vi "make 2D gaussian.vi"(9 "A":dbl=10.0, 10 "w":dbl=15.0) -> (0 "error out":errorcluster, 3 "LASER Pointing SYSTEM":dbl[][](graph))   [LabVIEW 2013]
uses:
  Interface/Non-General/BELLA/VIremote/VIremote.llb/VIremoteFunction.ctl
panel:
  in  "Next Button":bool
  in  "Previous Button":bool
  in  "Down Button":bool
  in  "Up Target":bool
  in  "error IO":errorcluster
  in  "Fire":bool
  out "Cursor.Cursor Position:Cursor Y":dbl
  out "Cursor.Cursor Position:Cursor X":dbl
  in  "Down":bool
  in  "Up":bool
  in  "Vertical":dbl
  in  "Right":bool
  in  "Left":bool
  in  "stop":bool
  in  "Horizontal":dbl
  out "#pix":dbl
  in  "No spot sizes 2":dbl=50.0 format="%.3f"
  out "x0":dbl=50.0
  in  "Ring":u16(ring)
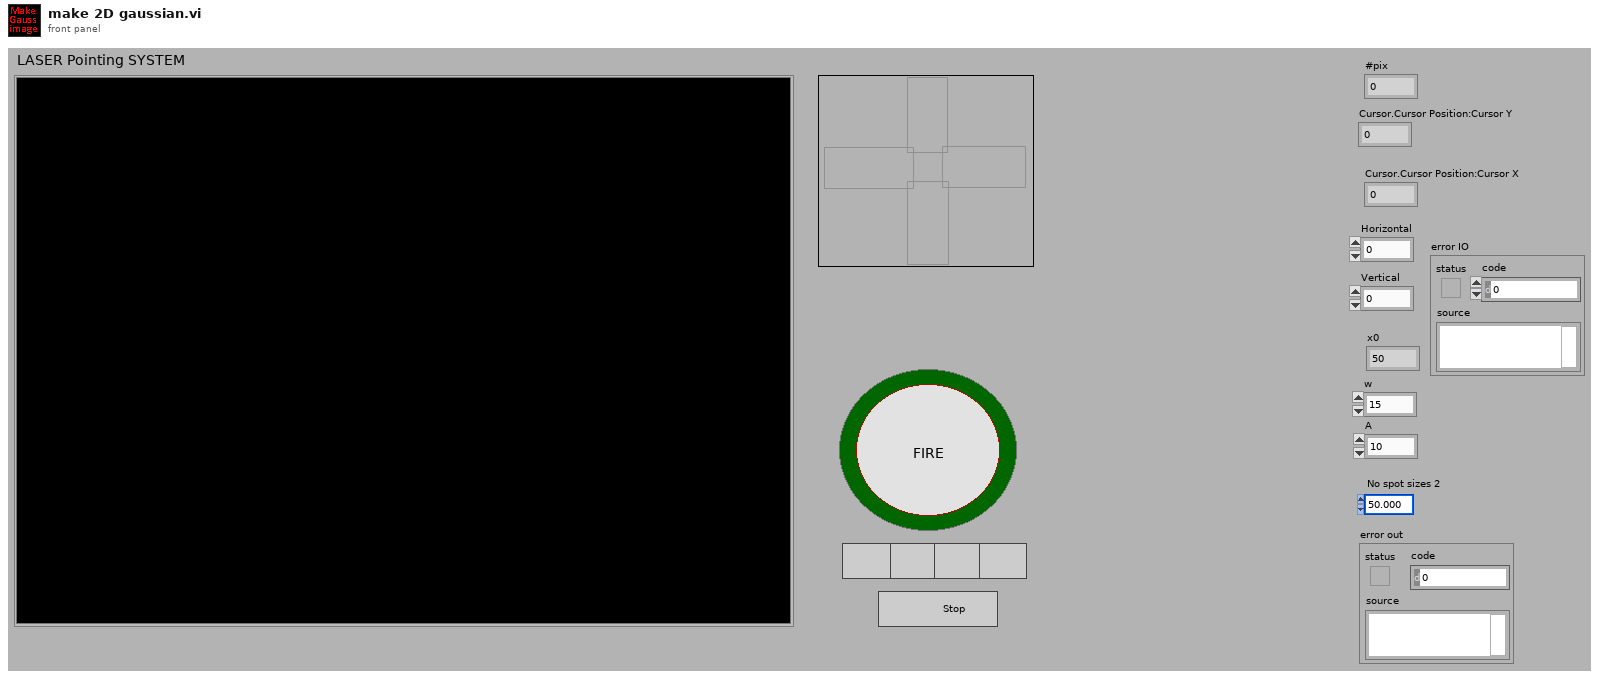
[diagram p1: front panel]
types:
  T1 = typedef "VIremoteFunction.ctl" = enum16{"Do nothing", "Stop controller", "Close this connection", "Show info panel", "Set VI to control", "Set Accelerometer freq (Hz)", "Show Alert message", "Start Sound Input", "Stop Sound Input", "Set Volume (0-100)", "Set sound output Speaker", "Set sound output Receiver", "Play Sound", "Repeat Sound", "Stop Sound", "Pause Sound", "Resume Sound", "Set panel width of caller (320 or 480)", "Set Panel Size to Portrait", "Set Panel Size to Landscape", "Set Panel Size as Current Orientation", "Allow all UI Orientations", "Send user notification", "Disable Scrolling", "Normal Scrolling", "Page Scrolling", "Set Scroll Offset", "Page Indicator Position"}
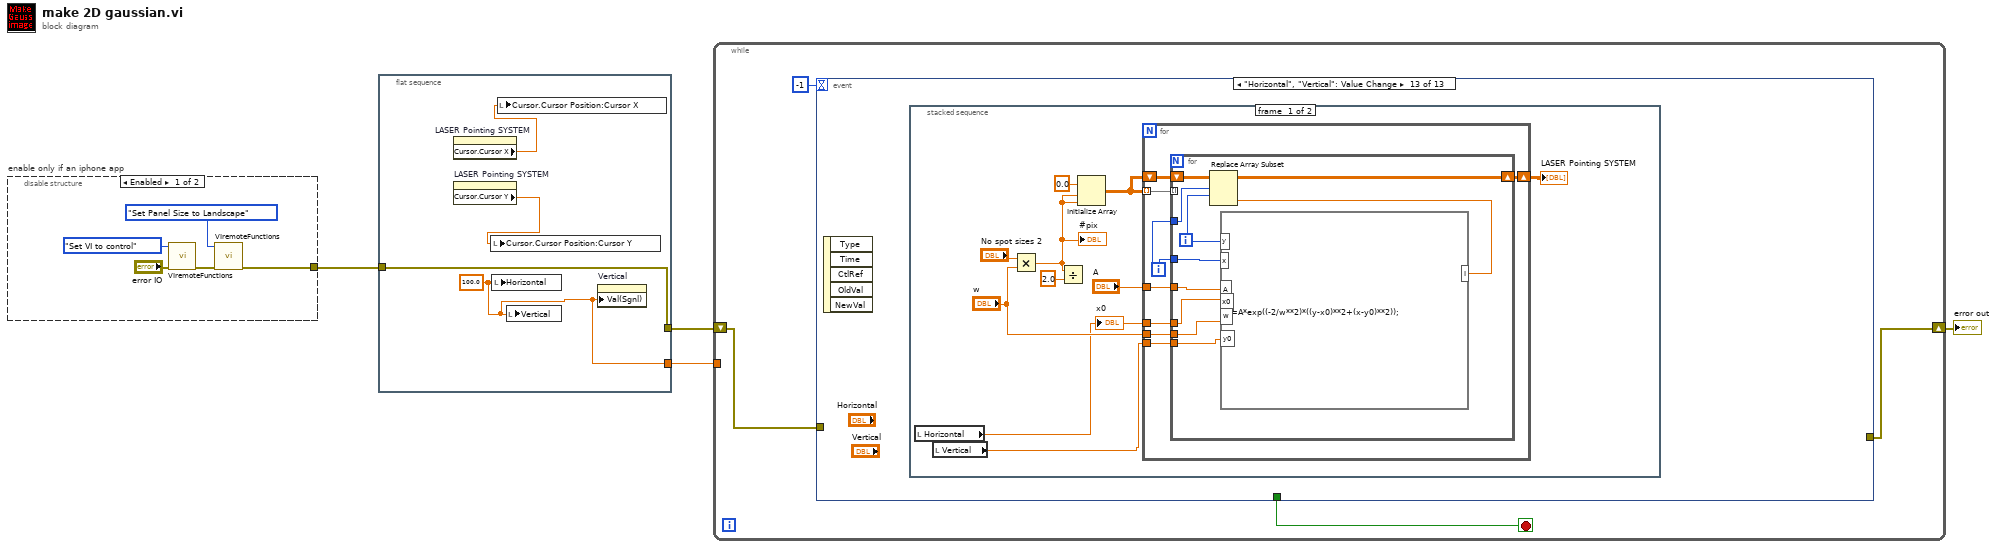
[diagram p0: block diagram]
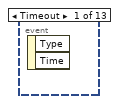
[diagram p3: hidden frame]
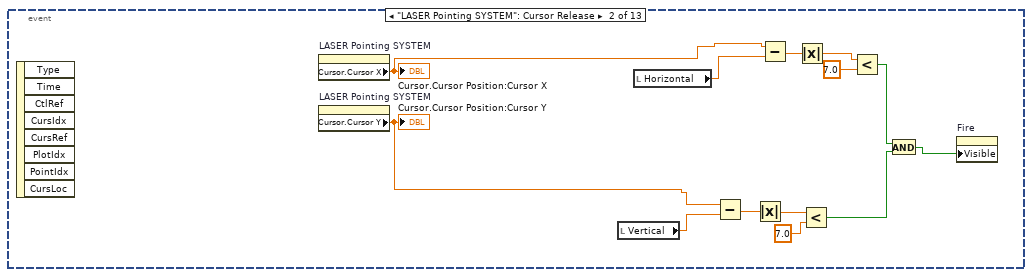
[diagram p4: hidden frame]
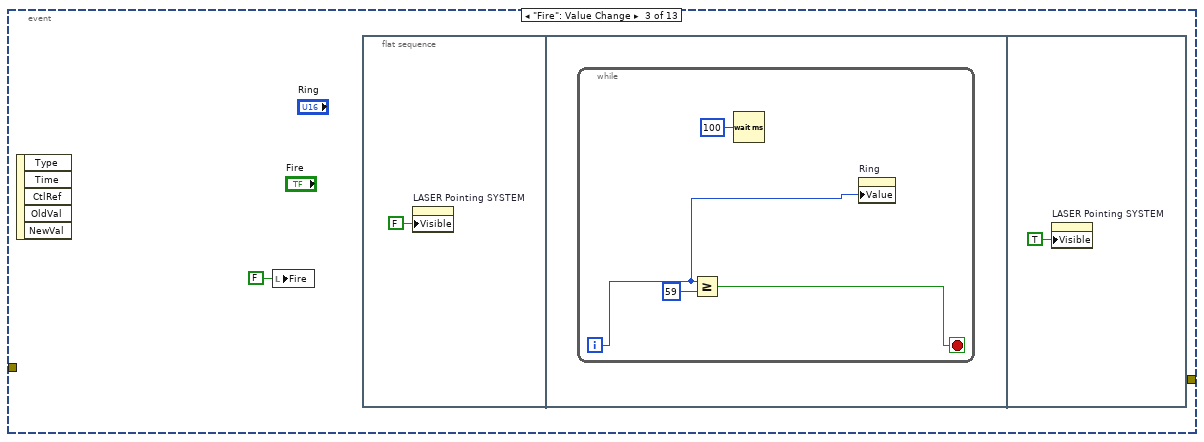
[diagram p5: hidden frame]
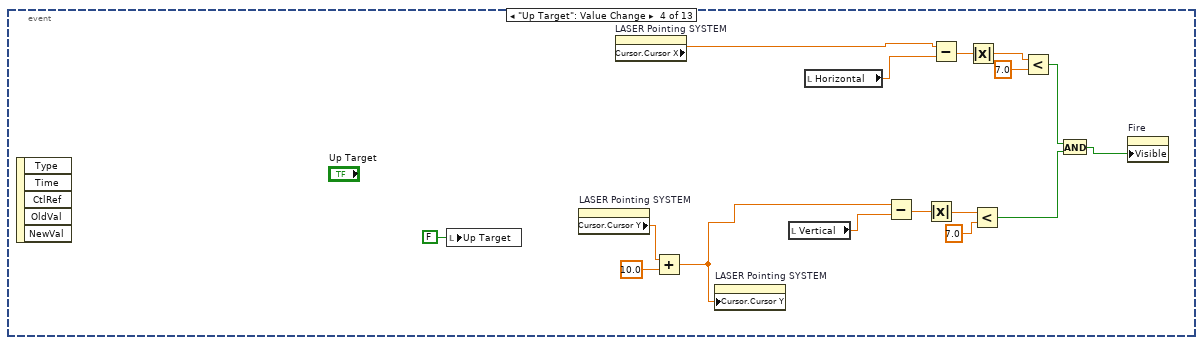
[diagram p6: hidden frame]
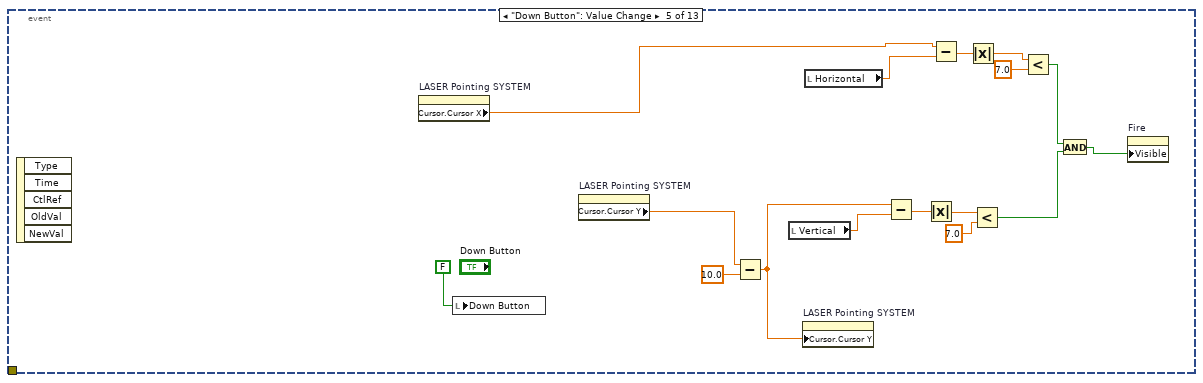
[diagram p7: hidden frame]
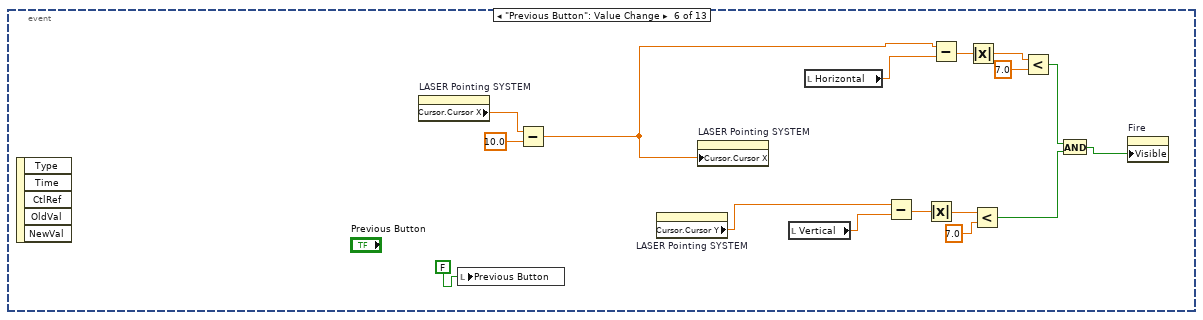
[diagram p8: hidden frame]
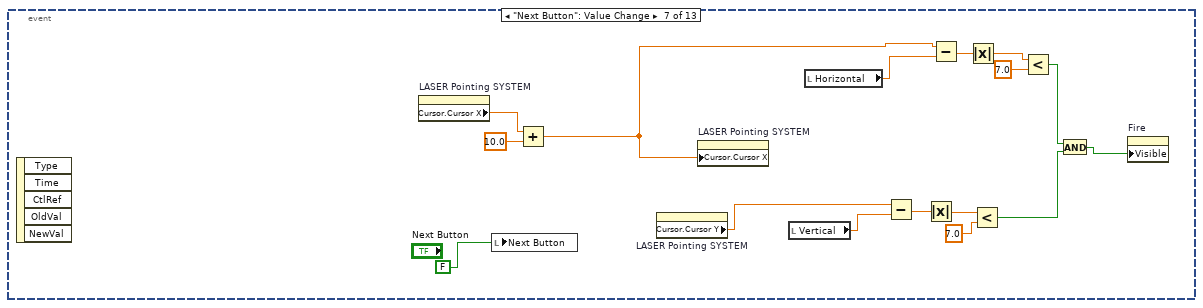
[diagram p9: hidden frame]
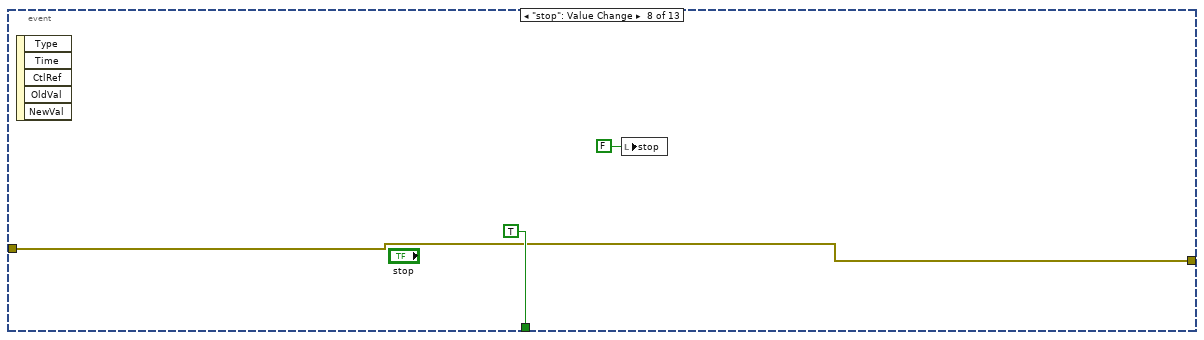
[diagram p10: hidden frame]
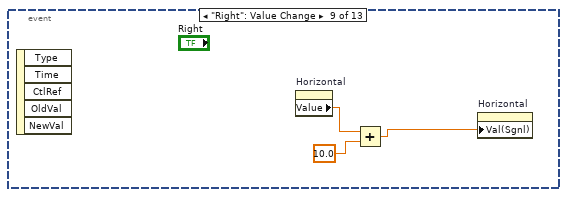
[diagram p11: hidden frame]
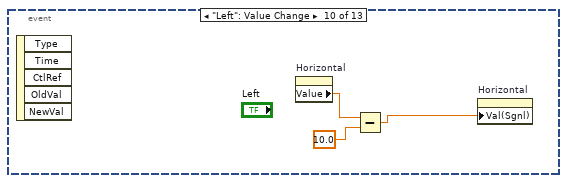
[diagram p12: hidden frame]
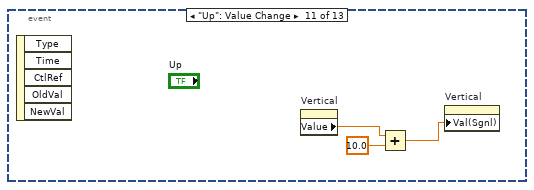
[diagram p13: hidden frame]
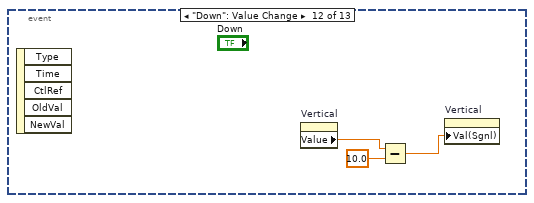
[diagram p14: hidden frame]
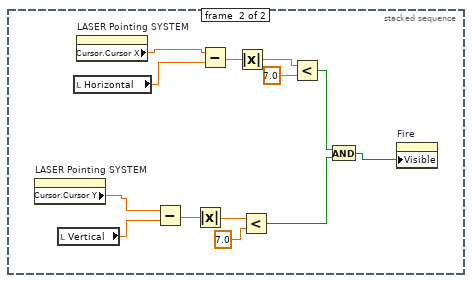
[diagram p15: hidden frame]
diagram:
  n1 = disable-structure "enable only if an iphone app" shown="Enabled" {
    disable-tunnel: [w5 _] -> w3
    frame Enabled {
      n2 = call "VIremoteFunctions.vi"("error in (no error)"="error IO", "Function"=VIremoteFunction."Set VI to control") -> ("error out"=w6:errorcluster)  [unwired: 4 in, 5 out]
      n3 = call "VIremoteFunctions.vi"("error in (no error)"=w6, "Function"=VIremoteFunction."Set Panel Size to Landscape") -> ("error out"=w5:errorcluster)  [unwired: 4 in, 5 out]
    }
    frame Disabled {
    }
  }
  n4 = flat-sequence {
    tunnel: [w13] -> w4
    tunnel: w3 -> [w10]
    tunnel: [w10] -> w2
    frame #0 {
      w13 = 100.0 ("Horizontal")
      n5 = property on="LASER Pointing SYSTEM" class="IntGraph (strict)"() -> ("Cursor.Cursor X"=w12:dbl)  [unwired: 2 in, 2 out]
      n6 = property on="LASER Pointing SYSTEM" class="IntGraph (strict)"() -> ("Cursor.Cursor Y"=w11:dbl)  [unwired: 2 in, 2 out]
      n7 = local write "Cursor.Cursor Position:Cursor Y"(w11) -> ()
      n8 = local write "Horizontal"(w13) -> ()
      n9 = local write "Cursor.Cursor Position:Cursor X"(w12) -> ()
      n10 = local write "Vertical"(w13) -> ()
      n11 = property on="Vertical" class="DigNum (strict)"("Val(Sgnl)"=w13) -> ()  [unwired: 2 in, 2 out]
    }
  }
  n12 = while {
    tunnel: w4 -> [_]
    shift-right: [w14] -> w1
    shift-left: w2 -> [w15]
    stop <- w17 stop-if-true
    n13 = event shown="[12] \"Horizontal\", \"Vertical\": Value Change" {
      selector: _ -> [_ _ _ _ _ _ _ _ _ _ _ _ _]
      dyn-events: _ -> [_ _ _ _ _ _ _ _ _ _ _ _ _]
      timeout: -1 -> [_ _ _ _ _ _ _ _ _ _ _ _ _]
      tunnel: [_ _ _ _ _ _ _ TRUE _ _ _ _ _] -> w17
      tunnel: w15 -> [_ _ _ _ _ _ _ w102 _ _ _ _ _]
      tunnel: [_ _ _ _ _ _ _ w102 _ _ _ _ _] -> w14
      event Timeout {
        n14 = event-data() -> ()  [unwired: 1 in, 2 out]
      }
      event "LASER Pointing SYSTEM": Cursor Release {
        n15 = event-data() -> ()  [unwired: 1 in, 8 out]
        n16 = property on="LASER Pointing SYSTEM" class="IntGraph (strict)"() -> ("Cursor.Cursor X"=w19:dbl)  [unwired: 2 in, 2 out]
        "Cursor.Cursor Position:Cursor X" <- w19
        n17 = property on="LASER Pointing SYSTEM" class="IntGraph (strict)"() -> ("Cursor.Cursor Y"=w18:dbl)  [unwired: 2 in, 2 out]
        "Cursor.Cursor Position:Cursor Y" <- w18
        n18 = local read "Vertical"() -> (w29:dbl)
        n19 = local read "Horizontal"() -> (w30:dbl)
        n20 = Subtract(x=w18, y=w29) -> (x-y=w27:dbl)
        n21 = Absolute Value(x=w27) -> (abs(x)=w24:dbl)
        n22 = Subtract(x=w19, y=w30) -> (x-y=w28:dbl)
        n23 = Absolute Value(x=w28) -> (abs(x)=w26:dbl)
        n24 = Less?(x=w24, y=7.0) -> (x < y?=w22:bool)
        n25 = Less?(x=w26, y=7.0) -> (x < y?=w21:bool)
        n26 = And(x=w21, y=w22) -> (x .and. y?=w20:bool)
        n27 = property on="Fire" class="Bool (strict)"("Visible"=w20) -> ()  [unwired: 2 in, 2 out]
      }
      event "Fire": Value Change {
        n28 = event-data() -> ()  [unwired: 1 in, 5 out]
        n29 = local write "Fire"(FALSE ("Fire")) -> ()
        n30 = flat-sequence {
          frame #0 {
            n31 = property on="LASER Pointing SYSTEM" class="IntGraph (strict)"("Visible"=FALSE) -> ()  [unwired: 2 in, 2 out]
          }
          frame #1 {
            n32 = while {
              i -> [w33]
              stop <- w35 stop-if-true
              n33 = Greater Or Equal?(x=w33, y=59) -> (x >= y?=w35:bool)
              n34 = Wait (ms)(milliseconds to wait=u32 100) -> ()  [unwired: 1 out]
              n35 = property on="Ring" class="Ring (strict)"("Value"=w33) -> ()  [unwired: 2 in, 2 out]
            }
          }
          frame #2 {
            n36 = property on="LASER Pointing SYSTEM" class="IntGraph (strict)"("Visible"=TRUE) -> ()  [unwired: 2 in, 2 out]
          }
        }
      }
      event "Up Target": Value Change {
        n37 = event-data() -> ()  [unwired: 1 in, 5 out]
        n38 = local write "Up Target"(FALSE ("Up Target")) -> ()
        n39 = property on="LASER Pointing SYSTEM" class="IntGraph (strict)"() -> ("Cursor.Cursor Y"=w40:dbl)  [unwired: 2 in, 2 out]
        n40 = property on="LASER Pointing SYSTEM" class="IntGraph (strict)"() -> ("Cursor.Cursor X"=w39:dbl)  [unwired: 2 in, 2 out]
        n41 = Add(x=w40, y=10.0) -> (x+y=w38:dbl)
        n42 = property on="LASER Pointing SYSTEM" class="IntGraph (strict)"("Cursor.Cursor Y"=w38) -> ()  [unwired: 2 in, 2 out]
        n43 = local read "Vertical"() -> (w51:dbl)
        n44 = local read "Horizontal"() -> (w52:dbl)
        n45 = Subtract(x=w38, y=w51) -> (x-y=w49:dbl)
        n46 = Absolute Value(x=w49) -> (abs(x)=w46:dbl)
        n47 = Subtract(x=w39, y=w52) -> (x-y=w50:dbl)
        n48 = Absolute Value(x=w50) -> (abs(x)=w48:dbl)
        n49 = Less?(x=w46, y=7.0) -> (x < y?=w44:bool)
        n50 = Less?(x=w48, y=7.0) -> (x < y?=w43:bool)
        n51 = And(x=w43, y=w44) -> (x .and. y?=w42:bool)
        n52 = property on="Fire" class="Bool (strict)"("Visible"=w42) -> ()  [unwired: 2 in, 2 out]
      }
      event "Down Button": Value Change {
        n53 = event-data() -> ()  [unwired: 1 in, 5 out]
        n54 = property on="LASER Pointing SYSTEM" class="IntGraph (strict)"() -> ("Cursor.Cursor X"=w54:dbl)  [unwired: 2 in, 2 out]
        n55 = local write "Down Button"(FALSE ("Down Button")) -> ()
        n56 = property on="LASER Pointing SYSTEM" class="IntGraph (strict)"() -> ("Cursor.Cursor Y"=w56:dbl)  [unwired: 2 in, 2 out]
        n57 = Subtract(x=w56, y=10.0) -> (x-y=w55:dbl)
        n58 = local read "Vertical"() -> (w67:dbl)
        n59 = property on="LASER Pointing SYSTEM" class="IntGraph (strict)"("Cursor.Cursor Y"=w55) -> ()  [unwired: 2 in, 2 out]
        n60 = local read "Horizontal"() -> (w68:dbl)
        n61 = Subtract(x=w55, y=w67) -> (x-y=w65:dbl)
        n62 = Absolute Value(x=w65) -> (abs(x)=w62:dbl)
        n63 = Subtract(x=w54, y=w68) -> (x-y=w66:dbl)
        n64 = Absolute Value(x=w66) -> (abs(x)=w64:dbl)
        n65 = Less?(x=w62, y=7.0) -> (x < y?=w60:bool)
        n66 = Less?(x=w64, y=7.0) -> (x < y?=w59:bool)
        n67 = And(x=w59, y=w60) -> (x .and. y?=w58:bool)
        n68 = property on="Fire" class="Bool (strict)"("Visible"=w58) -> ()  [unwired: 2 in, 2 out]
      }
      event "Previous Button": Value Change {
        n69 = event-data() -> ()  [unwired: 1 in, 5 out]
        n70 = property on="LASER Pointing SYSTEM" class="IntGraph (strict)"() -> ("Cursor.Cursor X"=w85:dbl)  [unwired: 2 in, 2 out]
        n71 = local write "Previous Button"(FALSE ("Down Button")) -> ()
        n72 = Subtract(x=w85, y=10.0) -> (x-y=w72:dbl)
        n73 = property on="LASER Pointing SYSTEM" class="IntGraph (strict)"() -> ("Cursor.Cursor Y"=w71:dbl)  [unwired: 2 in, 2 out]
        n74 = property on="LASER Pointing SYSTEM" class="IntGraph (strict)"("Cursor.Cursor X"=w72) -> ()  [unwired: 2 in, 2 out]
        n75 = local read "Vertical"() -> (w82:dbl)
        n76 = local read "Horizontal"() -> (w83:dbl)
        n77 = Subtract(x=w71, y=w82) -> (x-y=w80:dbl)
        n78 = Absolute Value(x=w80) -> (abs(x)=w77:dbl)
        n79 = Subtract(x=w72, y=w83) -> (x-y=w81:dbl)
        n80 = Absolute Value(x=w81) -> (abs(x)=w79:dbl)
        n81 = Less?(x=w77, y=7.0) -> (x < y?=w75:bool)
        n82 = Less?(x=w79, y=7.0) -> (x < y?=w74:bool)
        n83 = And(x=w74, y=w75) -> (x .and. y?=w73:bool)
        n84 = property on="Fire" class="Bool (strict)"("Visible"=w73) -> ()  [unwired: 2 in, 2 out]
      }
      event "Next Button": Value Change {
        n85 = event-data() -> ()  [unwired: 1 in, 5 out]
        n86 = property on="LASER Pointing SYSTEM" class="IntGraph (strict)"() -> ("Cursor.Cursor X"=w101:dbl)  [unwired: 2 in, 2 out]
        n87 = local write "Next Button"(FALSE ("Down Button")) -> ()
        n88 = Add(x=w101, y=10.0) -> (x+y=w88:dbl)
        n89 = property on="LASER Pointing SYSTEM" class="IntGraph (strict)"() -> ("Cursor.Cursor Y"=w87:dbl)  [unwired: 2 in, 2 out]
        n90 = property on="LASER Pointing SYSTEM" class="IntGraph (strict)"("Cursor.Cursor X"=w88) -> ()  [unwired: 2 in, 2 out]
        n91 = local read "Vertical"() -> (w98:dbl)
        n92 = local read "Horizontal"() -> (w99:dbl)
        n93 = Subtract(x=w87, y=w98) -> (x-y=w96:dbl)
        n94 = Absolute Value(x=w96) -> (abs(x)=w93:dbl)
        n95 = Subtract(x=w88, y=w99) -> (x-y=w97:dbl)
        n96 = Absolute Value(x=w97) -> (abs(x)=w95:dbl)
        n97 = Less?(x=w93, y=7.0) -> (x < y?=w91:bool)
        n98 = Less?(x=w95, y=7.0) -> (x < y?=w90:bool)
        n99 = And(x=w90, y=w91) -> (x .and. y?=w89:bool)
        n100 = property on="Fire" class="Bool (strict)"("Visible"=w89) -> ()  [unwired: 2 in, 2 out]
      }
      event "stop": Value Change {
        n101 = event-data() -> ()  [unwired: 1 in, 5 out]
        n102 = local write "stop"(FALSE ("Stop")) -> ()
      }
      event "Right": Value Change {
        n103 = event-data() -> ()  [unwired: 1 in, 5 out]
        n104 = property on="Horizontal" class="DigNum (strict)"() -> ("Value"=w107:dbl)  [unwired: 2 in, 2 out]
        n105 = Add(x=w107, y=10.0) -> (x+y=w105:dbl)
        n106 = property on="Horizontal" class="DigNum (strict)"("Val(Sgnl)"=w105) -> ()  [unwired: 2 in, 2 out]
      }
      event "Left": Value Change {
        n107 = event-data() -> ()  [unwired: 1 in, 5 out]
        n108 = property on="Horizontal" class="DigNum (strict)"() -> ("Value"=w110:dbl)  [unwired: 2 in, 2 out]
        n109 = Subtract(x=w110, y=10.0) -> (x-y=w108:dbl)
        n110 = property on="Horizontal" class="DigNum (strict)"("Val(Sgnl)"=w108) -> ()  [unwired: 2 in, 2 out]
      }
      event "Up": Value Change {
        n111 = event-data() -> ()  [unwired: 1 in, 5 out]
        n112 = property on="Vertical" class="DigNum (strict)"() -> ("Value"=w113:dbl)  [unwired: 2 in, 2 out]
        n113 = Add(x=w113, y=10.0) -> (x+y=w112:dbl)
        n114 = property on="Vertical" class="DigNum (strict)"("Val(Sgnl)"=w112) -> ()  [unwired: 2 in, 2 out]
      }
      event "Down": Value Change {
        n115 = event-data() -> ()  [unwired: 1 in, 5 out]
        n116 = property on="Vertical" class="DigNum (strict)"() -> ("Value"=w116:dbl)  [unwired: 2 in, 2 out]
        n117 = Subtract(x=w116, y=10.0) -> (x-y=w115:dbl)
        n118 = property on="Vertical" class="DigNum (strict)"("Val(Sgnl)"=w115) -> ()  [unwired: 2 in, 2 out]
      }
      event "Horizontal", "Vertical": Value Change {
        n119 = event-data() -> ()  [unwired: 1 in, 5 out]
        n120 = stacked-sequence {
          frame #0 {
            n121 = local read "Horizontal"() -> (w117:dbl)
            "x0" <- w117
            n122 = local read "Vertical"() -> (w118:dbl)
            n123 = Multiply(x="No spot sizes 2", y="w") -> (x*y=w123:dbl)
            "#pix" <- w123
            n124 = Divide(x=w123, y=2.0) -> ()  [unwired: 1 out]
            n125 = Initialize Array(0.0 ("element"), w123, w123) -> (w120:dbl[][])
            n126 = for {
              tunnel: w120 -> [w134] mode=indexing
              shift-right: [w132] -> w125
              shift-left: w120 -> [w133]
              tunnel: "A" -> [w131]
              tunnel: w117 -> [w129]
              tunnel: "w" -> [w128]
              tunnel: w118 -> [w127]
              i -> [w130]
              n127 = for {
                tunnel: w134 -> [_] mode=indexing
                shift-right: [w143] -> w132
                shift-left: w133 -> [w144]
                tunnel: w130 -> [w142]
                tunnel: w131 -> [w139]
                tunnel: w130 -> [w138]
                tunnel: w129 -> [w137]
                tunnel: w128 -> [w136]
                tunnel: w127 -> [w135]
                i -> [w141]
                n128 = formula code="I=A*exp((-2/w**2)*((y-x0)**2+(x-y0)**2));"("y"=w141, "A"=w139, "x0"=w137, "x"=w138, "w"=w136, "y0"=w135) -> ("I"=w140:dbl)
                n129 = Replace Array Subset(array=w144, new element=w140, index (row)=w142, index (col)=w141) -> (w143:dbl[][])
              }
            }
            "LASER Pointing SYSTEM" <- w125
          }
          frame #1 {
            n130 = property on="LASER Pointing SYSTEM" class="IntGraph (strict)"() -> ("Cursor.Cursor Y"=w155:dbl)  [unwired: 2 in, 2 out]
            n131 = local read "Vertical"() -> (w154:dbl)
            n132 = local read "Horizontal"() -> (w156:dbl)
            n133 = property on="LASER Pointing SYSTEM" class="IntGraph (strict)"() -> ("Cursor.Cursor X"=w157:dbl)  [unwired: 2 in, 2 out]
            n134 = Subtract(x=w155, y=w154) -> (x-y=w152:dbl)
            n135 = Absolute Value(x=w152) -> (abs(x)=w149:dbl)
            n136 = Subtract(x=w157, y=w156) -> (x-y=w153:dbl)
            n137 = Absolute Value(x=w153) -> (abs(x)=w151:dbl)
            n138 = Less?(x=w149, y=7.0) -> (x < y?=w147:bool)
            n139 = Less?(x=w151, y=7.0) -> (x < y?=w146:bool)
            n140 = And(x=w146, y=w147) -> (x .and. y?=w145:bool)
            n141 = property on="Fire" class="Bool (strict)"("Visible"=w145) -> ()  [unwired: 2 in, 2 out]
          }
        }
      }
    }
  }
  "error out" <- w1
